vi "NewUI2.vi"() -> ()   [LabVIEW 2012]
panel:
  in  "Brightness":i32(slide) min=0 max=100 step=1 scale=0.0..100.0
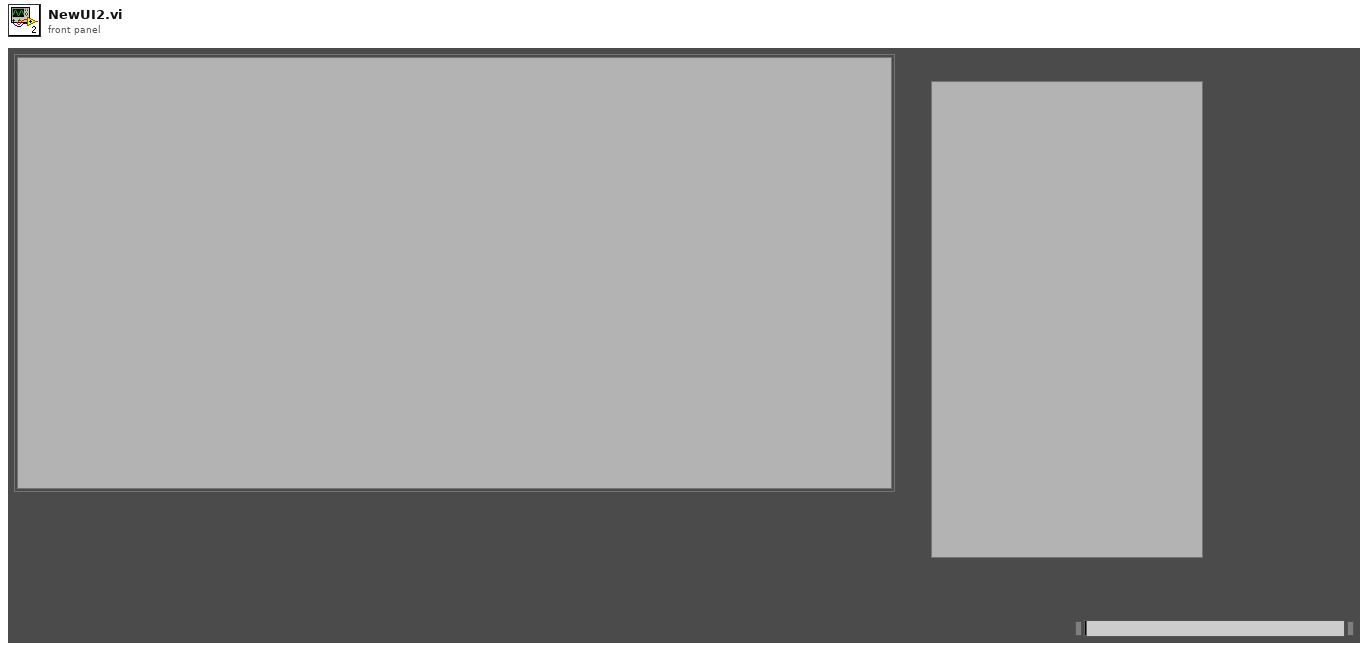
[diagram p1: front panel]
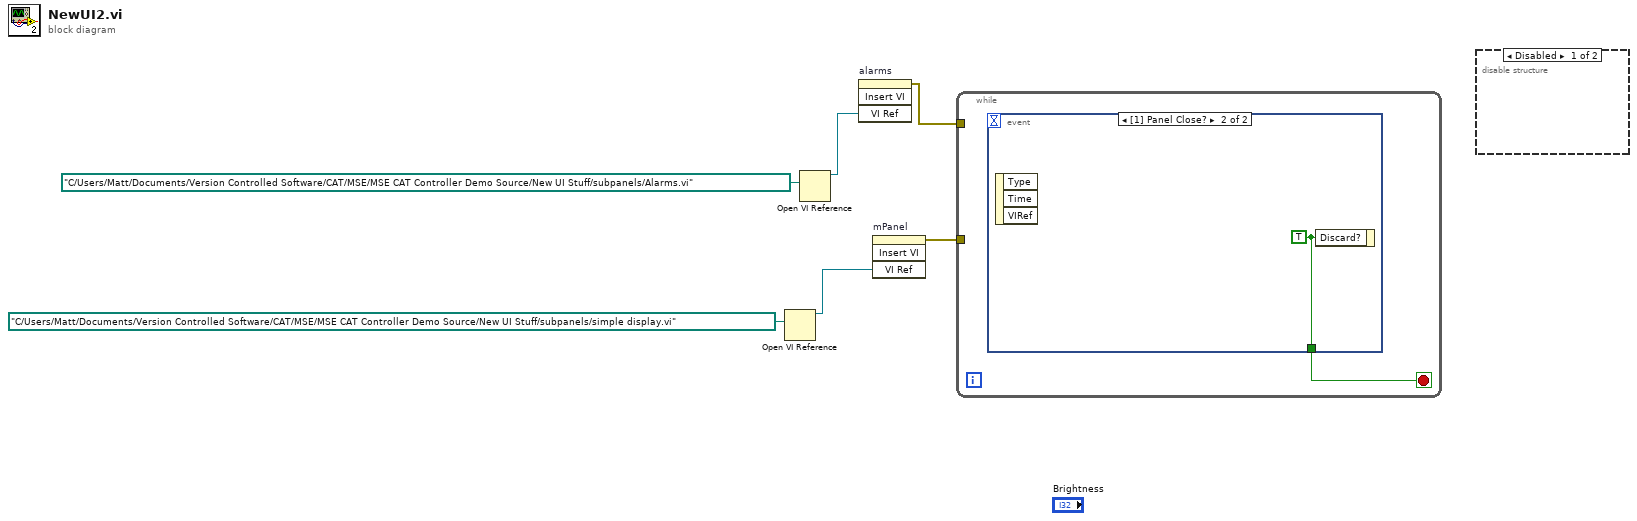
[diagram p0: block diagram]
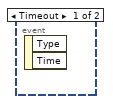
[diagram p3: hidden frame]
diagram:
  n1 = Open VI Reference(vi path=path "C:/Users/Matt/Documents/Version Controlled Software/CAT/MSE/MSE CAT Controller Demo Source/New UI Stuff/subpanels/simple display.vi") -> (vi reference=w2:refnum<vi>)  [unwired: 5 in, 1 out]
  n2 = Open VI Reference(vi path=path "C:/Users/Matt/Documents/Version Controlled Software/CAT/MSE/MSE CAT Controller Demo Source/New UI Stuff/subpanels/Alarms.vi") -> (vi reference=w5:refnum<vi>)  [unwired: 5 in, 1 out]
  n3 = invoke on="alarms" class="SubPanel" method="Insert VI"("VI Ref"=w5) -> (error out=w4:errorcluster)  [unwired: 3 in, 3 out]
  n4 = invoke on="mPanel" class="SubPanel" method="Insert VI"("VI Ref"=w2) -> (error out=w1:errorcluster)  [unwired: 3 in, 3 out]
  n5 = while {
    tunnel: w4 -> [_]
    tunnel: w1 -> [_]
    stop <- w7 stop-if-true
    n6 = event shown="[1] Panel Close?" {
      selector: _ -> [_ _]
      dyn-events: _ -> [_ _]
      timeout: _ -> [_ _]
      tunnel: [_ w8] -> w7
      event Timeout {
        n7 = event-data() -> ()  [unwired: 1 in, 2 out]
      }
      event Panel Close? {
        w8 = TRUE ("Discard?")
        n8 = event-data() -> ()  [unwired: 1 in, 3 out]
        n9 = event-data("Discard?"=w8) -> ()  [unwired: 1 in, 1 out]
      }
    }
  }
  n10 = disable-structure shown="Disabled" {
    frame Disabled {
    }
    frame Enabled {
    }
  }
